vi "UHR-Fleezers Control (host) - 10.5.vi"() -> ()   [LabVIEW 2010] (continued)
    tunnel: "Initial Phase Adj. (MCL)" -> [w275]
    tunnel: w144 -> [w276]
    tunnel: w145 -> [w277]
    tunnel: "Initial Phase Adjustment (GI)" -> [w278]
    tunnel: "Initial Phase Adjustment (AI1)" -> [w279]
    tunnel: [w279] -> w8
    tunnel: [w278] -> w7
    tunnel: [w277] -> w6
    tunnel: [w276] -> w5
    tunnel: [w275] -> w4
    tunnel: [w274] -> w3
    tunnel: [w273] -> w2
    tunnel: [w291] -> w154
    tunnel: [w285] -> w150
    tunnel: "Initial Phase Adjustment (APD Acq)" -> [w284]
    tunnel: "Initial Phase Adjustment (APD 1 Gate)" -> [w283]
    tunnel: "Initial Phase Adjustment (Green FB)" -> [w282]
    tunnel: w8 -> [w290]
    tunnel: w7 -> [w289]
    tunnel: w6 -> [w288]
    tunnel: w5 -> [w287]
    tunnel: w4 -> [w286]
    tunnel: w3 -> [w281]
    tunnel: w2 -> [w280]
    tunnel: w154 -> [w470]
    tunnel: [w471] -> w151
    tunnel: w150 -> [w471]
    tunnel: [w470] -> w149
    tunnel: w151 -> [w474]
    tunnel: w149 -> [w473]
    tunnel: [w476] -> w148
    tunnel: [w475] -> w147
    tunnel: [w663] -> w152
    tunnel: [w664] -> w153
    tunnel: w148 -> [w664]
    tunnel: w147 -> [w663]
    frame #0 {
      n114 = Wait (ms)(milliseconds to wait=u32 200) -> ()  [unwired: 1 out]
    }
    frame #1 {
      n115 = xnode "Read/Write Control"("FPGA VI Reference In"=w288, "error in"=w287, "Phase count adjustment"=w290, "Phase count adjustment (GI)"=w289, "Phase count adjustment (MCL)"=w286, "Phase Count Adjustment (APD Acq)"=w284, "Phase count adjustment (APD 1 Gate)"=w283, "Phase count adjustment (APD 2 Gate)"=w280, "Phase count adjustment (Green FB)"=w282, "Phase count adjustment (GI) 2"=w281) -> ("FPGA VI Reference Out"=w285:T20, "error out"=w291:errorcluster)
    }
    frame #2 {
      n116 = Wait (ms)(milliseconds to wait=u32 200) -> ()  [unwired: 1 out]
    }
    frame #3 {
      w472 = TRUE
      n117 = xnode "Read/Write Control"("FPGA VI Reference In"=w474, "error in"=w473, "+ phase"=w472, "+ phase (GI)"=w472, "+ phase (MCL)"=w472, "+ phase (APD Acq)"=w472, "+ phase (APD 1 Gate)"=w472, "+ phase (APD 2 Gate)"=w472, "+ phase (Green FB)"=w472, "+ phase (GI) 2"=w472) -> ("FPGA VI Reference Out"=w475:T20, "error out"=w476:errorcluster)
    }
    frame #4 {
      n118 = Wait (ms)(milliseconds to wait=u32 200) -> ()  [unwired: 1 out]
    }
  }
  n119 = local read "Phase adj. (Green FB)"() -> (w118:i16)
  n120 = local read "Phase adj. (GI) 2"() -> (w88:i16)
  n121 = local read "Phase adjust (MCL)"() -> (w183:i16)
  n122 = local read "Phase adj. (AI1)"() -> (w185:i16)
  n123 = local read "Phase adj. (GI)"() -> (w184:i16)
  n124 = xnode "Read/Write Control"("FPGA VI Reference In"=w152, "error in"=w153, "Phase count adjustment"=w185, "Phase count adjustment (GI)"=w184, "Phase count adjustment (MCL)"=w183, "Phase Count Adjustment (APD Acq)"="Phase Adj. (APD Acq)", "Phase count adjustment (APD 1 Gate)"="Phase Adj. (APD 1 Gate)", "Phase count adjustment (APD 2 Gate)"="Phase Adj. (APD 2 Gate)", "Phase count adjustment (Green FB)"=w118, "Phase count adjustment (GI) 2"=w88) -> ("FPGA VI Reference Out"=w75:T20, "error out"=w161:errorcluster)
  n125 = call "Initialize RF boards - interlace 3.vi"("error in"=w161, "FPGA VI Reference In"=w75) -> ("error out"=w159:errorcluster, "FPGA VI Reference Out"=w160:T20)
  n126 = call "set RF board frequency - interlace.vi"("Board 2 Frequency Limits"=w121, "Board 1 Frequency Limits"=w123, "error in"=w159, "FPGA VI Reference In"=w160, "Board 2 Frequency 3 (MHz)"="BD 2 Frequency 3 (MHz)", "Board 1 Frequency 3 (MHz)"="BD 1 Frequency 3 (MHz)", "Board 2 Frequency 2 (MHz)"="BD 2 Frequency 2 (MHz)", "Board 2 Frequency 1 (MHz)"="BD 2 Frequency 1 (MHz)", "Board 1 Frequency 2 (MHz)"="BD 1 Frequency 2 (MHz)", "Board 1 Frequency 1  (MHz)"="BD 1 Frequency 1 (MHz)") -> ("error out"=w257:errorcluster, "FPGA VI Reference Out"=w258:T20)
  n127 = call "set RF board amplitude - interlace.vi"("Board 2 Amplitude Limits"=w120, "Board 1 Amplitude Limits"=w122, "error in"=w257, "FPGA VI Reference In"=w258, "Board 2 Amplitude 3 (%)"="BD 2 Amplitude 3 (%)", "Board 1 Amplitude 3 (%)"="BD 1 Amplitude 3 (%)", "Board 2 Amplitude 2 (%)"="BD 2 Amplitude 2 (%)", "Board 2 Amplitude 1 (%)"="BD 2 Amplitude 1 (%)", "Board 1 Amplitude 2 (%)"="BD 1 Amplitude 2 (%)", "Board 1 Amplitude 1 (%)"="BD 1 Amplitude 1 (%)") -> ("error out"=w245:errorcluster, "FPGA VI Reference Out"=w246:T20)
  n128 = flat-sequence {
    tunnel: w246 -> [w673]
    tunnel: w245 -> [w672]
    tunnel: [w671] -> w250
    tunnel: [w670] -> w249
    tunnel: [w715] -> w248
    tunnel: w250 -> [w715]
    tunnel: [w714] -> w247
    tunnel: w249 -> [w714]
    tunnel: w248 -> [w724]
    tunnel: w247 -> [w723]
    tunnel: [w722] -> w34
    tunnel: [w721] -> w33
    tunnel: [w780] -> w35
    tunnel: [w789] -> w9
    tunnel: w34 -> [w789]
    tunnel: w33 -> [w784]
    frame #0 {
      n129 = local read "Trap 1 (ON/OFF)"() -> (w665:bool)
      n130 = xnode "Read/Write Control"("FPGA VI Reference In"=w673, "error in"=w672, "Direct RF Box  Communication"=FALSE) -> ("FPGA VI Reference Out"=w671:T20, "error out"=w670:errorcluster)
      n131 = local write "Saving..."(FALSE ("Saving Data")) -> ()
      n132 = local write "Stop All"(FALSE ("Stop All")) -> ()
      n133 = local write "Index"(1.0 ("Index")) -> ()
      n134 = property on="Trap 1 ON" class="Bool (strict)"("Value"=w665) -> ()  [unwired: 2 in, 2 out]
      "Manipulating Trap" <- FALSE ("Manipulating Trap")
    }
    frame #1 {
      n135 = local read "Trap 2 (ON/OFF)"() -> (w713:bool)
      n136 = Wait (ms)(milliseconds to wait=u32 50) -> ()  [unwired: 1 out]
      n137 = property on="Trap 2 ON" class="Bool (strict)"("Val(Sgnl)"=w713) -> ()  [unwired: 2 in, 2 out]
    }
    frame #2 {
      n138 = local read "Scan Range (nm)"() -> (w717:dbl)
      n139 = xnode "Read/Write Control"("FPGA VI Reference In"=w724, "error in"=w723, "FPGA Controls  RF Box"=TRUE ("Direct RF Box  Communication")) -> ("FPGA VI Reference Out"=w722:T20, "error out"=w721:errorcluster)
      n140 = call "Update messages.vi"("Message to add"="UHR-Fleezers ready.", "Old message string"="") -> ("New message string"=w720:string)
      n141 = local write "Messages"(w720) -> ()
      n142 = property on="Scan Range (nm)" class="DigNum (strict)"("Val(Sgnl)"=w717) -> ()  [unwired: 2 in, 2 out]
    }
    frame #3 {
      w769 = T23."ASCII" ("Command")
      # "disable hysteresis\ncompensation for\nfaster performance"
      # "increase jerk\nfor faster \nresponse"
      # "disable backlash\ncompensation for\nfaster response \ntimes. necessary\nfor mouse control\nof stage"
      n143 = call "CONEX_FUNCTIONAL_GLOBAL.vi"("error in"=w784, "Command"=T23."INIT") -> ("error out"=w765:errorcluster)  [unwired: 7 in, 2 out]
      n144 = call "CONEX_FUNCTIONAL_GLOBAL.vi"("error in"=w765, "Position"=dbl[] [10.0, 12.0, 6.2], "Command"=T23."SET ULIM") -> ("error out"=w785:errorcluster)  [unwired: 6 in, 2 out]
      n145 = call "CONEX_FUNCTIONAL_GLOBAL.vi"("error in"=w785, "Position"=dbl[] [4.0, 0.0, 5.8], "Command"=T23."SET LLIM") -> ("error out"=w778:errorcluster)  [unwired: 6 in, 2 out]
      n146 = Concatenate Strings("1BA0", "\r\n") -> (w775:string)
      n147 = call "CONEX_FUNCTIONAL_GLOBAL.vi"("error in"=w778, "ASCII command"=w775, "Command"=w769) -> ("error out"=w774:errorcluster)  [unwired: 6 in, 2 out]
      n148 = Concatenate Strings("1JR0.001", "\r\n") -> (w771:string)
      n149 = call "CONEX_FUNCTIONAL_GLOBAL.vi"("error in"=w774, "ASCII command"=w771, "Command"=w769) -> ("error out"=w770:errorcluster)  [unwired: 6 in, 2 out]
      n150 = Concatenate Strings("1BH0", "\r\n") -> (w766:string)
      n151 = call "CONEX_FUNCTIONAL_GLOBAL.vi"("error in"=w770, "ASCII command"=w766, "Command"=w769) -> ("error out"=w764:errorcluster)  [unwired: 6 in, 2 out]
      n152 = call "CONEX_FUNCTIONAL_GLOBAL.vi"("error in"=w764, "Command"=T23."GET POS") -> ("error out"=w780:errorcluster, "Current Position"=w779:dbl[])  [unwired: 7 in, 1 out]
      n153 = local write "Current Position"(w779) -> ()
    }
  }
  n154 = Subtract(x="BD 1 Frequency 1 (MHz)", y="BD 1 Frequency 2 (MHz)") -> (x-y=w171:dbl)
  n155 = Subtract(x="BD 2 Frequency 1 (MHz)", y="BD 2 Frequency 2 (MHz)") -> (x-y=w170:dbl)
  n156 = Square(x=w170) -> (x^2=w168:dbl)
  n157 = Square(x=w171) -> (x^2=w169:dbl)
  n158 = Add(x=w169, y=w168) -> (x+y=w167:dbl)
  n159 = Square Root(x=w167) -> (sqrt(x)=w166:dbl)
  n160 = local write "Trap Delta (MHz)"(w166) -> ()
  n161 = call "IMAQ Create"("Image Name"="APD 1 Image", "Image Type"=w66) -> ("New Image"=w65:T2)  [unwired: 3 in, 1 out]
  n162 = call "IMAQ Create"("Image Name"="APD 2 Image", "Image Type"=w66) -> ("New Image"=w64:T2)  [unwired: 3 in, 1 out]
  n163 = call "IMAQ Create"("Image Name"="Det. X Image", "Image Type"=w66) -> ("New Image"=w63:T2)  [unwired: 3 in, 1 out]
  n164 = call "IMAQ Create"("Image Name"="Det. Y Image", "Image Type"=w66) -> ("New Image"=w62:T2)  [unwired: 3 in, 1 out]
  n165 = call-poly "VISA Configure Serial Port"("VISA resource name"="Harvard Syringe Pump Serial Port", "baud rate (9600)"=u32 115200, "stop bits (10: 1 bit)"=w59) -> ("VISA resource name out"=w56:refnum<visa-resource-name>, "error out"=w57:errorcluster)  [unwired: 4 in, 7 out]
  n166 = Bundle("New Image"=w65, "New Image"=w64, "New Image"=w63, "New Image"=w62) -> (w61:T24)  [unwired: 1 in]
  n167 = Tick Count (ms)() -> (millisecond timer value=w36:u32)
  n168 = call <vilib>:"IMAQ Init.vi"("Interface Name"="img0") -> ("error out"=w28:errorcluster, "IMAQ Session Out"=w30:refnum<k11>)  [unwired: 9 in]
  n169 = disable-structure shown="Disabled" {
    disable-tunnel: w9 -> [w792 _]
    frame Disabled {
      n170 = call <vilib>:"Initialize Mouse.vi"() -> ("device ID"=w791:refnum<k1>)  [unwired: 10 in, 1 out]
      n171 = while {
        tunnel: w792 -> [_]
        tunnel: w791 -> [w796]
        tunnel: [w795] -> w790
        stop <- w794 stop-if-true
        n172 = event shown="[2] \"Use mouse to move stage\n(press any key to quit)\": Value Change" {
          selector: _ -> [_ _ _ _]
          dyn-events: _ -> [_ _ _ _]
          timeout: 1 -> [_ _ _ _]
          tunnel: w796 -> [w797 w798 w808 _]
          tunnel: [w797 w798 w804 _] -> w795
          tunnel: [_ w799 _ _] -> w794
          event Timeout {
            n173 = event-data() -> ()  [unwired: 1 in, 2 out]
          }
          event "Stop All": Value Change {
            n174 = event-data() -> ()  [unwired: 1 in, 5 out]
            n175 = local read "Stop All"() -> (w799:bool)
          }
          event "Use mouse to move stage\n(press any key to quit)": Value Change {
            n176 = event-data() -> ()  [unwired: 1 in, 1 out]
            n177 = local write "Stage Moving"(TRUE ("Stage Moving")) -> ()
            n178 = call-poly <vilib>:"Acquire Input Data.vi"("device ID"=w808) -> ("device ID"=w805:refnum<k1>)  [unwired: 15 in, 3 out]
            n179 = node-c288() -> (w807:T25)  [unwired: 4 in]
            n180 = timed-loop {
              timing: w807 -> [_]
              timing-out: [_] -> w806
              tunnel: w805 -> [w838]
              tunnel: [w837] -> w804
              tunnel: [w810] -> w801
              stop <- w813 stop-if-true
              (unwired) 10
              # "put cursor somewhere\nwhere mouse clicks and \nmouse wheel moves won't\nbe heard by the window"
              # "SetCursorPos"
              n181 = node-c288() -> ()  [unwired: 1 in, 1 out]
              n182 = call-poly <vilib>:"Acquire Input Data.vi"("device ID"=w838, "key mode"=enum16{"RELATIVE", "ABSOLUTE"}."RELATIVE") -> ("device ID"=w837:refnum<k1>, "axis info"=w835:T28, "button info"=w825:T29)  [unwired: 14 in, 1 out]
              n183 = Cluster To Array(cluster=w835) -> (array=w833:i32[])
              n184 = Unbundle By Name(w825) -> ("button 1"=w824:bool, "button 2"=w823:bool, "button 3"=w822:bool)
              n185 = Compound Arithmetic op=MULTIPLY(invert 10000.0 ("value"), "mouse sensitivity", w833) -> (w831:dbl[])
              n186 = call "subVI_explode3array.vi"("Array"=w831) -> ("x"=w817:dbl, "y"=w816:dbl, "z"=w830:dbl)  [unwired: 12 in]
              n187 = case shown="False" "invert y?" {
                tunnel: w816 -> [w839 w841]
                tunnel: [w839 w840] -> w815
                frame False {
                }
                frame True {
                  n188 = Negate(x=w841) -> (-x=w840:dbl)
                }
              }
              n189 = case shown="False" "invert x?" {
                tunnel: w817 -> [w842 w844]
                tunnel: [w842 w843] -> w814
                frame False {
                }
                frame True {
                  n190 = Negate(x=w844) -> (-x=w843:dbl)
                }
              }
              n191 = Compound Arithmetic op=OR(w824, w823, w822) -> (w813:bool)
              n192 = Divide(x=w830, y=50.0) -> (x/y=w828:dbl)
              n193 = Build Array(w814, w815, w828) -> (w820:dbl[])
              n194 = Not(x=w813) -> (.not. x?=w821:bool)
              n195 = call "CONEX_FUNCTIONAL_GLOBAL.vi"("Axis"=enum16{"X", "Y", "Z", "XY", "XZ", "YZ", "XYZ"}."XYZ", "Position"=w820, "Command"=T23."REL MOVE") -> ("error out"=w810:errorcluster)  [unwired: 6 in, 2 out]
              n196 = dll-call lib="User32.dll" fn="SetCursorPos"(700, 45) -> ()  [unwired: 5 in, 3 out]
              n197 = local write "Stage Moving"(w821) -> ()
              n198 = node-c288() -> ()  [unwired: 1 in, 1 out]
            }
            n199 = node-c288(w806) -> ()  [unwired: 1 out]
            n200 = call "CONEX_FUNCTIONAL_GLOBAL.vi"("Axis"=enum16{"X", "Y", "Z", "XY", "XZ", "YZ", "XYZ"}."XYZ", "error in"=w801, "Command"=T23."GET POS") -> ("Current Position"=w800:dbl[])  [unwired: 6 in, 2 out]
            n201 = local write "Current Position"(w800) -> ()
          }
          event "reset motor comm. link": Value Change {
            n202 = event-data() -> ()  [unwired: 1 in, 1 out]
          }
        }
      }
      n203 = call-poly <vilib>:"Close Input Device.vi"("device ID"=w790) -> ()  [unwired: 9 in, 1 out]
    }
    frame Enabled {
    }
  }
  n204 = call <vilib>:"IMAQ Grab Setup.vi"("error in (no error)"=w28, "IMAQ Session In"=w30) -> ("error out"=w24:errorcluster, "IMAQ Session Out"=w25:refnum<k11>)  [unwired: 8 in]
  n205 = call "IMAQ Create"("Image Name"="untitled", "Image Type"=w26) -> ("New Image"=w23:T2)  [unwired: 3 in, 1 out]
  n206 = node-c288() -> (w32:T25)  [unwired: 4 in]
  n207 = timed-loop "acquire video and stage position" {
    timing: w32 -> [_]
    timing-out: [_] -> w31
    tunnel: w25 -> [w859]
    tunnel: w24 -> [w858]
    tunnel: w23 -> [w857]
    tunnel: [w856] -> w20
    tunnel: [w853] -> w19
    tunnel: [w854] -> w18
    tunnel: w9 -> [_]
    shift-right: [w850] -> _
    shift-left: cluster{i32, i32, i32, i32}[] [] -> [w851]
    stop <- w855 stop-if-true
    n208 = node-c288() -> ()  [unwired: 1 in, 1 out]
    n209 = event shown="[2] \"Primary Video Display\": Mouse Down" {
      selector: _ -> [_ _ _ _]
      dyn-events: _ -> [_ _ _ _]
      timeout: 10 -> [_ _ _ _]
      tunnel: w859 -> [w870 w885 w893 w913]
      tunnel: w858 -> [w869 w887 w891 w915]
      tunnel: w857 -> [w868 w886 w892 w914]
      tunnel: [w867 w885 w893 w913] -> w856
      tunnel: [w860 w889 FALSE FALSE] -> w855
      tunnel: [w864 w887 w891 w915] -> w854
      tunnel: [w863 w886 w892 w914] -> w853
      tunnel: "radius" -> [_ _ w899 _]
      tunnel: w851 -> [w861 w888 w897 _]
      tunnel: [w861 w888 w898 cluster{i32, i32, i32, i32}[] []] -> w850
      event Timeout {
        n210 = event-data() -> ()  [unwired: 1 in, 2 out]
        n211 = call <vilib>:"IMAQ Grab Acquire.vi"("error in (no error)"=w869, "Image In"=w868, "IMAQ Session In"=w870) -> ("error out"=w865:errorcluster, "Image Out"=w866:T2, "IMAQ Session Out"=w867:refnum<k11>)  [unwired: 5 in, 1 out]
        n212 = case shown="True" "trap\nmarkers?" {
          tunnel: w861 -> [_ w878]
          tunnel: w866 -> [w872 w877]
          tunnel: w865 -> [w871 w876]
          tunnel: [w871 w875] -> w864
          tunnel: [w872 w873] -> w863
          frame False {
          }
          frame True {
            n213 = for {
              tunnel: w878 -> [w884] mode=indexing
              shift-right: [w882] -> w873
              shift-left: w877 -> [w883]
              tunnel: w876 -> [w881]
              tunnel: [w880] -> w875
              tunnel: u32 16711680 ("Color") -> [w879]
              n214 = call "IMAQ Overlay Oval"("Color"=w879, "error in (no error)"=w881, "Bounding Rectangle"=w884, "Image"=w883) -> ("error out"=w880:errorcluster, "Image Out"=w882:T2)  [unwired: 6 in]
            }
          }
        }
        "Primary Video Display" <- w863
        n215 = Unbundle By Name(w865) -> ("status"=w860:bool)
      }
      event "Stop All": Value Change {
        n216 = event-data() -> ()  [unwired: 1 in, 5 out]
        n217 = local read "Stop All"() -> (w889:bool)
      }
      event "Primary Video Display": Mouse Down {
        n218 = event-data() -> ()  [unwired: 1 in, 7 out]
        n219 = Array Size(array=w897) -> (size(s)=w896:i32)
        n220 = Less?(x=w896, y=2) -> (x < y?=w894:bool)
        n221 = case shown="True" w894 {
          tunnel: w899 -> [_ w909]
          tunnel: w897 -> [w900 w903]
          tunnel: [w900 w902] -> w898
          frame False {
          }
          frame True {
            n222 = property on="Primary Video Display" class="ImageControl"() -> ("Last Mouse Position"=w901:cluster{"X":i32, "Y":i32})  [unwired: 2 in, 2 out]
            n223 = Unbundle By Name(w901) -> ("X"=w911:i32, "Y"=w910:i32)
            n224 = Add(x=w910, y=w909) -> (x+y=w907:i32)
            n225 = Subtract(x=w910, y=w909) -> (x-y=w905:i32)
            n226 = Add(x=w911, y=w909) -> (x+y=w906:i32)
            n227 = Subtract(x=w911, y=w909) -> (x-y=w908:i32)
            n228 = Bundle(w908, w907, w906, w905) -> (w904:cluster{i32, i32, i32, i32})  [unwired: 1 in]
            n229 = Build Array (concatenate)(w903, w904) -> (w902:cluster{i32, i32, i32, i32}[])
          }
        }
      }
      event "clear markers": Value Change {
        n230 = event-data() -> ()  [unwired: 1 in, 5 out]
      }
    }
    n231 = node-c288() -> ()  [unwired: 1 in, 1 out]
    "Array" <- w851
  }
  n232 = node-c288(i64 1 ("Period"), 1 ("Processor")) -> (w175:T25)  [unwired: 2 out]
  n233 = node-c288(2 ("Processor")) -> (w79:T25)  [unwired: 3 out]
  n234 = node-c288() -> (w71:T25)  [unwired: 4 in]
  n235 = node-c288() -> (w81:T25)  [unwired: 4 out]
  n236 = timed-loop "Acquire Data" {
    tunnel: w9 -> [w1175]
    tunnel: w35 -> [w1174]
    tunnel: [w1205] -> w11
    tunnel: [w1199] -> w10
    timing: w175 -> [_]
    timing-out: [_] -> w174
    tunnel: w61 -> [w1003]
    shift-right: [w920] -> _
    shift-left: w36 -> [w922]
    stop <- "Stop All" stop-if-true
    (unwired) u32 0 ("Number of Elements")
    w990 = "NI_ChannelName" ("name")
    # "originally this was Trap AI FIFO Depth -\nTrap AI Elements/DMA read. The subtraction\nof zero is a kluge to make it work."
    n237 = node-c288() -> ()  [unwired: 2 out]
    n238 = Tick Count (ms)() -> (millisecond timer value=w920:u32)
    n239 = First Call?() -> (First Call?: T/F=w956:bool)
    n240 = Subtract(x=w920, y=w922) -> (x-y=→"x-y":u32)
    n241 = Or(x="Reset", y=w956) -> (x .or. y?=w957:bool)
    n242 = case "Reset data stream" shown="True" w957 {
      tunnel: w1175 -> [w1219 w1227]
      tunnel: w1174 -> [w1218 w1226]
      tunnel: [w1219 w1221] -> w1170
      tunnel: [w1218 w1220] -> w1169
      frame False {
      }
      frame True {
        w1224 = TRUE ("AI to FIFO")
        n243 = local write "Overflow (data lost)"(FALSE ("Overflow (data lost)")) -> ()
        n244 = call "reset FPGA DMA.vi"("error in"=w1226, "FPGA VI Reference In"=w1227) -> ("error out"=w1222:errorcluster, "FPGA VI Reference Out"=w1223:T20)
        n245 = xnode "Read/Write Control"("FPGA VI Reference In"=w1223, "error in"=w1222, "AI to FIFO"=w1224, "APD to FIFO"=w1224) -> ("FPGA VI Reference Out"=w1221:T20, "error out"=w1220:errorcluster)
      }
    }
    n246 = Or(x="Start AOD Scan", y="Trap Raster Scan") -> (x .or. y?=w1120:bool)
    n247 = case "Start AOM raster scan" shown="False" w1120 {
      tunnel: w1170 -> [w2835 w2845]
      tunnel: w1169 -> [w2834 w2844]
      tunnel: [w2835 w2838] -> w1168
      tunnel: [w2834 w2837] -> w1167
      frame False {
      }
      frame True {
        n248 = case shown="True" "Restart DMA? (AOD)" {
          tunnel: [w3256 w3258] -> w2839
          tunnel: [w3255 w3257] -> w2840
          tunnel: w2845 -> [w3256 w3260]
          tunnel: w2844 -> [w3255 w3259]
          frame False {
          }
          frame True {
            n249 = local write "Overflow (data lost)"(FALSE ("Overflow (data lost)")) -> ()
            n250 = call "reset FPGA DMA.vi"("error in"=w3259, "FPGA VI Reference In"=w3260) -> ("error out"=w3257:errorcluster, "FPGA VI Reference Out"=w3258:T20)
          }
        }
        n251 = local write "Trap Raster Scan"(FALSE ("Trap Raster Scan")) -> ()
        n252 = case shown="True" "Move MCL Also?" {
          tunnel: w2840 -> [w2848 w2957]
          tunnel: w2839 -> [w2849 w2958]
          tunnel: [w2847 w2961] -> w2838
          tunnel: [w2846 w2960] -> w2837
          frame False {
            w2850 = TRUE ("AI to FIFO")
            n253 = xnode "Read/Write Control"("FPGA VI Reference In"=w2849, "error in"=w2848, "AI to FIFO"=w2850, "APD to FIFO"=w2850, "Start scan"=w2850) -> ("FPGA VI Reference Out"=w2847:T20, "error out"=w2846:errorcluster)
          }
          frame True {
            w2954 = FALSE ("1D or 2D Scan?")
            w2959 = TRUE ("AI to FIFO")
            # "Count for MCL loop"
            # "N total cycles"
            # "N steps"
            # "V_int"
            n254 = local read "Scan Range (nm)"() -> (w2936:dbl)
            n255 = local read "Number of F/B Scans (AOD)"() -> (w2953:u16)
            n256 = Sign(1:w2936) -> (0:w2935:dbl)
            n257 = Compound Arithmetic op=MULTIPLY(w2936, "MCL Step Position Ratio", "MCL/AOM Scale Tweak") -> (w2940:dbl)
            n258 = Negate(x=w2935) -> (-x=w2932:dbl)
            n259 = Multiply(x=w2932, y="MCL Step Increment (V_int)") -> (x*y=w2934:dbl)
            n260 = Divide(x=w2940, y="MCL X Cal (nm/V)") -> (x/y=w2946:dbl)
            n261 = Multiply(x=32767.0 ("y"), y=w2946) -> (x*y=w2952:dbl)
            n262 = local read "Total Counts (ticks)"() -> (w2937:u32)
            n263 = local read "Cycles/step (AOD)"() -> (w2948:u64)
            n264 = local read "Scan steps (AOD)"() -> (w2949:u64)
            n265 = Divide(x=w2952, y=10.0) -> (x/y=w2945:dbl)
            n266 = Divide(x=w2945, y="MCL Step Increment (V_int)") -> (x/y=w2943:dbl)
            n267 = Absolute Value(x=w2943) -> (abs(x)=w2931:dbl)
            n268 = Compound Arithmetic op=MULTIPLY(w2949, w2948, w2937) -> (w2944:u64)
            n269 = local write "wait to reset values"(w2959) -> ()
            n270 = local write "MCL Scanning"(w2959) -> ()
            n271 = Divide(x=w2944, y=w2931) -> (x/y=w2941:dbl)
            "MCL Count" <- w2941
            n272 = xnode "Read/Write Control"("FPGA VI Reference In"=w2958, "error in"=w2957, "Scan steps (MCL)"=w2931, "Number of scans (MCL)"=w2953, "Cycles per step (MCL)"=u64 1, "Scan freq.  increment (MCL)"=w2934, "1D or 2D Scan?"=w2954, "MCL Scan Axis"=w2954, "Cont. Scan (MCL)"=w2954, "MCL count"=w2941) -> ("FPGA VI Reference Out"=w2956:T20, "error out"=w2955:errorcluster)
            n273 = xnode "Read/Write Control"("FPGA VI Reference In"=w2956, "error in"=w2955, "AI to FIFO"=w2959, "APD to FIFO"=w2959, "Start scan"=w2959, "Start scan (MCL)"=w2959) -> ("FPGA VI Reference Out"=w2961:T20, "error out"=w2960:errorcluster)
          }
        }
        "Raster Scanning..." <- TRUE ("Scanning...")
      }
    }
    n274 = And(x="Save scans", y=w1120) -> (x .and. y?=w1166:bool)
    n275 = Compound Arithmetic op=OR("Start MCL Scan", "Confocal Image", "Confocal Linescan") -> (w1118:bool)
    n276 = And(x="Save Data (MCL)", y=w1118) -> (x .and. y?=w1165:bool)
    n277 = case "Start MCL raster scan" shown="False" w1118 {
      tunnel: w1168 -> [w2176 w2191]
      tunnel: w1167 -> [w2175 w2190]
      tunnel: [w2176 w2186] -> w924
      tunnel: [w2175 w2185] -> w923
      tunnel: [FALSE w2184] -> w1151
      tunnel: "Start MCL Scan" -> [_ w2179]
      tunnel: "Confocal Image" -> [_ w2178]
      tunnel: "Confocal Linescan" -> [_ _]
      frame False {
      }
      frame True {
        w2184 = TRUE
        n278 = case shown="True" "Restart DMA? (MCL)" {
          tunnel: [w2436 w2438] -> w2189
          tunnel: [w2435 w2437] -> w2188
          tunnel: w2191 -> [w2436 w2441]
          tunnel: w2190 -> [w2435 w2440]
          frame False {
          }
          frame True {
            n279 = call "reset FPGA DMA.vi"("error in"=w2440, "FPGA VI Reference In"=w2441) -> ("error out"=w2437:errorcluster, "FPGA VI Reference Out"=w2438:T20)
            n280 = local write "Overflow (data lost)"(FALSE ("Overflow (data lost)")) -> ()
          }
        }
        n281 = case shown="False" w2179 {
          selector: w2179 -> [_ w2195]
          tunnel: w2178 -> [w2194 _]
          tunnel: [w2194 w2195] -> w2177
          frame False {
            n282 = property on="2D or 1D Scan" class="Bool (strict)"("Val(Sgnl)"=w2194) -> ()  [unwired: 2 in, 2 out]
            n283 = property on="Confocal Image" class="Bool (strict)"("Value"=FALSE ("Start Confocal Map")) -> ()  [unwired: 2 in, 2 out]
          }
          frame True {
          }
        }
        n284 = local write "MCL Scanning"(w2184) -> ()
        n285 = local read "AO1"() -> (w2181:dbl)
        n286 = local read "AO2"() -> (w2180:dbl)
        n287 = case shown="False" "Center Scan" {
          tunnel: w2189 -> [w2202 w2314]
          tunnel: w2188 -> [w2201 w2313]
          tunnel: [w2200 w2312] -> w2186
          tunnel: [w2199 w2311] -> w2185
          tunnel: [w2197 w2298] -> w2183
          tunnel: [w2196 w2297] -> w2182
          tunnel: w2181 -> [w2197 w2303]
          tunnel: w2180 -> [w2196 w2306]
          tunnel: w2177 -> [_ _]
          frame False {
            w2198 = TRUE ("AI to FIFO")
            n288 = xnode "Read/Write Control"("FPGA VI Reference In"=w2202, "error in"=w2201, "AI to FIFO"=w2198, "APD to FIFO"=w2198, "Start scan (MCL)"=w2198) -> ("FPGA VI Reference Out"=w2200:T20, "error out"=w2199:errorcluster)
          }
          frame True {
            w2310 = TRUE ("AI to FIFO")
            n289 = local read "Scan steps (MCL)"() -> (w2289:u64)
            n290 = local read "Scan lines (y)"() -> (w2285:u64)
            n291 = local read "Fast Scan Dir"() -> (w2296:bool)
            n292 = local read "Actual MCL Inc (V)"() -> (w2286:dbl)
            n293 = Decrement(x=w2285) -> (x-1=w2284:u64)
            n294 = Decrement(x=w2289) -> (x-1=w2288:u64)
            n295 = Multiply(x=w2286, y=w2284) -> (x*y=w2283:dbl)
            n296 = Divide(x=w2283, y=2.0) -> (x/y=w2293:dbl)
            n297 = Multiply(x=w2286, y=w2288) -> (x*y=w2287:dbl)
            n298 = Divide(x=w2287, y=2.0) -> (x/y=w2292:dbl)
            n299 = Select(t=w2292, s=w2296, f=w2293) -> (s? t:f=w2291:dbl)
            n300 = Select(t=w2293, s=w2296, f=w2292) -> (s? t:f=w2295:dbl)
            n301 = Subtract(x=w2303, y=w2295) -> (x-y=w2294:dbl)
            n302 = Subtract(x=w2306, y=w2291) -> (x-y=w2290:dbl)
            n303 = local read "2D or 1D Scan"() -> (w2308:bool)
            n304 = Not(x=w2296) -> (.not. x?=w2302:bool)
            n305 = Not(x=w2308) -> (.not. x?=w2304:bool)
            n306 = And(x=w2296, y=w2304) -> (x .and. y?=w2305:bool)
            n307 = And(x=w2304, y=w2302) -> (x .and. y?=w2307:bool)
            n308 = Select(t=w2306, s=w2307, f=w2290) -> (s? t:f=w2297:dbl)
            n309 = Select(t=w2303, s=w2305, f=w2294) -> (s? t:f=w2298:dbl)
            n310 = call "Volt to I16.vi"("Voltage In"=w2298) -> ("I16 Voltage Out"=w2301:i16)
            n311 = call "Volt to I16.vi"("Voltage In"=w2297) -> ("I16 Voltage Out"=w2300:i16)
            n312 = xnode "Read/Write Control"("FPGA VI Reference In"=w2314, "error in"=w2313, "AI to FIFO"=w2310, "APD to FIFO"=w2310, "Start scan (MCL)"=w2310, "AO1"=w2301, "AO2"=w2300) -> ("FPGA VI Reference Out"=w2312:T20, "error out"=w2311:errorcluster)
          }
        }
        "Initial Y" <- w2183
        "Initial X" <- w2182
        "wait to reset values" <- w2184
      }
    }
    n313 = local read "Trap Pos Elements/DMA read"() -> (w999:u32)
    n314 = local read "Trap AI Elements/DMA read"() -> (w919:u32)
    n315 = local read "APD Elements/DMA read"() -> (w1042:u32)
    n316 = local read "Trap AI FIFO Depth"() -> (w1215:u32)
    n317 = xnode "Get APD Data"("FPGA VI Reference In"=w924, "error in"=w923, "Number of Elements"=w1042, "Timeout (ms)"=-1) -> ("Data"=w1041:u32[], "Elements Remaining"=→"APD FIFO Elements Remaining":u32)  [unwired: 2 out]
    n318 = xnode "Invoke Method"("FPGA VI Reference In"=w924, "error in"=w923, "Number of Elements"=w999, "Timeout (ms)"=-1) -> ("Data"=w963:u16[], "Elements Remaining"=→"Trap Pos FIFO El Remaining":u32)  [unwired: 2 out]
    n319 = xnode "Invoke Method"("FPGA VI Reference In"=w924, "error in"=w923, "Number of Elements"=w919, "Timeout (ms)"=-1 ("Timeout")) -> ("FPGA VI Reference Out"=w926:T20, "error out"=w925:errorcluster, "Data"=w928:i16[], "Elements Remaining"=w927:u32)
    "Trap AI FIFO El. Rem." <- w927
    n320 = Subtract(x=w1215, y=w919) -> (x-y=w1214:u32)
    n321 = Decimate 1D Array(w963) -> (w960:u16[], w962:u16[], w961:u16[])
    n322 = Divide(x=w927, y=w1214) -> (x/y=w1213:dbl)
    "Buffer Status" <- w1213
    n323 = To Unsigned Long Integer(number=w960) -> (unsigned 32bit integer=w959:u32[])
    n324 = Join Numbers(hi=w962, lo=w961) -> ((hi.lo)=w958:u32[])
    n325 = Equal?(x=w1213, y=1.0) -> (x = y?=w1211:bool)
    n326 = Join Numbers(hi=w959, lo=w958) -> ((hi.lo)=w952:u64[])
    n327 = call "IR AOM word to freq - vec.vi"("Frequency Word In (double vec)"=w952) -> ("Frequency Out"=w998:dbl[])
    n328 = case "Alert buffer overflow" shown="True" w1211 {
      frame False {
      }
      frame True {
        n329 = call <vilib>:"Beep.vi"() -> ()  [unwired: 3 in, 9 out]
        "Overflow (data lost)" <- TRUE ("Overflow (data lost)")
      }
    }
    n330 = Decimate 1D Array(w998) -> (w997:dbl[], w996:dbl[])
    n331 = Build Array(w997, w996) -> (w995:dbl[][])
    n332 = local read "Trap Sets"() -> (w1079:u32)
    n333 = case "Deinterlace trap data, average down PSD" shown="2" w1079 {
      tunnel: w928 -> [w2471 w2536]
      tunnel: [w2468 w2533] -> w1072
      tunnel: [w2471 w2535] -> w955
      tunnel: "Detector Type" -> [w2470 w2531]
      tunnel: [w2469 w2534] -> w1071
      tunnel: [w2467 w2532] -> w1186
      frame 1, Default {
        n334 = Divide(x=w2471, y=3276.7) -> (x/y=w2472:dbl[])
        n335 = Decimate 1D Array(w2472) -> (w2481:dbl[], w2480:dbl[], w2479:dbl[], w2478:dbl[], w2477:dbl[], w2476:dbl[], w2475:dbl[], w2474:dbl[])
        n336 = case shown="\"IR-QPD + PSD + FB-QPD position\"" w2470 {
          tunnel: w2481 -> [w2505 w2530]
          tunnel: w2480 -> [w2504 w2529]
          tunnel: w2479 -> [w2489 w2507]
          tunnel: w2478 -> [w2490 w2517]
          tunnel: w2477 -> [w2503 w2528]
          tunnel: w2476 -> [w2502 w2527]
          tunnel: w2475 -> [w2486 w2508]
          tunnel: w2474 -> [w2485 w2506]
          tunnel: [w2484 w2514] -> w2469
          tunnel: [w2483 w2513] -> w2468
          tunnel: [w2482 w2512] -> w2467
          frame "IR-QPD + PSD + FB-QPD", Default {
            w2482 = 0  # Channel pattern
            n337 = Divide(x=w2505, y=w2490) -> (x/y=w2492:dbl[])
            n338 = Divide(x=w2504, y=w2490) -> (x/y=w2491:dbl[])
            n339 = Divide(x=w2503, y=w2486) -> (x/y=w2488:dbl[])
            n340 = Divide(x=w2502, y=w2485) -> (x/y=w2487:dbl[])
            n341 = Build Array(w2492, w2491, w2490, w2489, w2488, w2487, w2486, w2485) -> (w2483:dbl[][])
            n342 = Bundle("T1 Y", "T1 X", "T1 Sum", "FB Sum", "PSD Y", "PSD X", "PSD Y Sum", "PSD X Sum") -> (w2501:T39)  [unwired: 1 out]
            n343 = Cluster To Array(cluster=w2501) -> (array=w2484:string[])
          }
          frame "IR-QPD + PSD + FB-QPD position" {
            w2512 = 3  # Channel pattern
            n344 = Negate(x=w2508) -> (-x=w2509:dbl[])
            n345 = Divide(x=w2530, y=w2517) -> (x/y=w2519:dbl[])
            n346 = Divide(x=w2529, y=w2517) -> (x/y=w2518:dbl[])
            n347 = Divide(x=w2528, y=w2508) -> (x/y=w2516:dbl[])
            n348 = Divide(x=w2527, y=w2509) -> (x/y=w2515:dbl[])
            n349 = Build Array(w2519, w2518, w2517, w2506, w2507, w2516, w2515, w2508) -> (w2513:dbl[][])
            n350 = Bundle("T1 Y", "T1 X", "T1 Sum", "FB X", "FB Sum", "PSD Y", "PSD X", "PSD Y Sum") -> (w2526:T39)  [unwired: 1 out]
            n351 = Cluster To Array(cluster=w2526) -> (array=w2514:string[])
          }
        }
      }
      frame 2 {
        n352 = case shown="\"IR-QPD + PSD + FB-QPD X position\"" w2531 {
          tunnel: w2536 -> [w2598 w2665 w2736]
          tunnel: [w2537 w2656 w2667] -> w2535
          tunnel: [w2564 w2647 w2714] -> w2534
          tunnel: [w2563 w2610 w2681] -> w2533
          tunnel: [w2557 w2645 w2712] -> w2532
          frame "IR-QPD + PSD + FB-QPD", Default {
            w2557 = 1  # Channel pattern
            # "time average x2 the 4th signal and the 4 psd signals (detection laser)"
            # "deinterlace 3 signals from qpd"
            n353 = Decimate 1D Array(w2598) -> (w2597:i16[], w2596:i16[], w2562:i16[], w2595:i16[], w2585:i16[], w2583:i16[], w2582:i16[], w2580:i16[])
            n354 = Decimate 1D Array(w2562) -> (w2561:i16[], w2560:i16[])
            n355 = Decimate 1D Array(w2597) -> (w2594:i16[], w2566:i16[])
            n356 = Decimate 1D Array(w2596) -> (w2593:i16[], w2591:i16[])
            n357 = Decimate 1D Array(w2595) -> (w2592:i16[], w2590:i16[])
            n358 = call "downsample 1D array - double.vi"("Ave N"=2.0, "Array In"=w2585) -> ("Array Out"=w2584:dbl[])  [unwired: 1 out]
            n359 = call "downsample 1D array - double.vi"("Ave N"=2.0, "Array In"=w2583) -> ("Array Out"=w2565:dbl[])  [unwired: 1 out]
            n360 = call "downsample 1D array - double.vi"("Ave N"=2.0, "Array In"=w2582) -> ("Array Out"=w2581:dbl[])  [unwired: 1 out]
            n361 = call "downsample 1D array - double.vi"("Ave N"=2.0, "Array In"=w2580) -> ("Array Out"=w2579:dbl[])  [unwired: 1 out]
            n362 = Interleave 1D Arrays(w2594, w2593, w2592, w2566, w2591, w2590, w2561, w2560, w2584, w2565, w2581, w2579) -> (w2578:dbl[])
            n363 = Divide(x=w2578, y=3276.7) -> (x/y=w2577:dbl[])
            n364 = Decimate 1D Array(w2577) -> (w2576:dbl[], w2575:dbl[], w2574:dbl[], w2573:dbl[], w2572:dbl[], w2571:dbl[], w2559:dbl[], w2558:dbl[], w2570:dbl[], w2569:dbl[], w2568:dbl[], w2567:dbl[])
            n365 = Divide(x=w2576, y=w2574) -> (x/y=w2544:dbl[])
            n366 = Divide(x=w2575, y=w2574) -> (x/y=w2543:dbl[])
            n367 = Divide(x=w2573, y=w2571) -> (x/y=w2542:dbl[])
            n368 = Divide(x=w2572, y=w2571) -> (x/y=w2541:dbl[])
            n369 = Divide(x=w2570, y=w2568) -> (x/y=w2540:dbl[])
            n370 = Divide(x=w2569, y=w2567) -> (x/y=w2539:dbl[])
            n371 = Build Array(w2544, w2543, w2574, w2542, w2541, w2571, w2559, w2558, w2540, w2539, w2568, w2567) -> (w2563:dbl[][])
            n372 = Bundle("T1 Y", "T1 X", "T1 Sum", "T2 Y", "T2 X", "T2 Sum", "T1 FB Sum", "T2 FB Sum", "PSD Y", "PSD X", "PSD Y Sum", "PSD X Sum") -> (w2545:T40)  [unwired: 1 out]
            n373 = To Word Integer(number=w2578) -> (16bit integer=w2537:i16[])
            n374 = Cluster To Array(cluster=w2545) -> (array=w2564:string[])
          }
          frame "IR-QPD + PSD + FB-QPD X position" {
            w2645 = 2  # Channel pattern
            # "time average x2 the 3 psd signals (detection laser)"
            # "deinterlace 3 signals from qpds"
            n375 = Decimate 1D Array(w2665) -> (w2664:i16[], w2663:i16[], w2646:i16[], w2662:i16[], w2608:i16[], w2605:i16[], w2602:i16[], w2633:i16[])
            n376 = Decimate 1D Array(w2646) -> (w2631:i16[], w2629:i16[])
            n377 = Decimate 1D Array(w2664) -> (w2661:i16[], w2648:i16[])
            n378 = Decimate 1D Array(w2663) -> (w2660:i16[], w2658:i16[])
            n379 = Decimate 1D Array(w2662) -> (w2659:i16[], w2657:i16[])
            n380 = Decimate 1D Array(w2633) -> (w2632:i16[], w2630:i16[])
            n381 = call "downsample 1D array - I16.vi"("Ave N"=2.0, "Array In"=w2608) -> ("Array Out"=w2606:i16[])  [unwired: 1 in]
            n382 = call "downsample 1D array - I16.vi"("Ave N"=2.0, "Array In"=w2602) -> ("Array Out"=w2600:i16[])  [unwired: 1 in]
            n383 = call "downsample 1D array - I16.vi"("Ave N"=2.0, "Array In"=w2605) -> ("Array Out"=w2603:i16[])  [unwired: 1 in]
            n384 = Interleave 1D Arrays(w2661, w2660, w2659, w2648, w2658, w2657, w2632, w2631, w2630, w2629, w2606, w2603, w2600) -> (w2656:i16[])
            n385 = Divide(x=w2656, y=3276.7) -> (x/y=w2655:dbl[])
            n386 = Decimate 1D Array(w2655) -> (w2654:dbl[], w2653:dbl[], w2652:dbl[], w2651:dbl[], w2650:dbl[], w2649:dbl[], w2621:dbl[], w2619:dbl[], w2618:dbl[], w2616:dbl[], w2615:dbl[], w2614:dbl[], w2611:dbl[])
            n387 = Negate(x=w2611) -> (-x=w2609:dbl[])
            n388 = Divide(x=w2615, y=w2611) -> (x/y=w2613:dbl[])
            n389 = Divide(x=w2614, y=w2609) -> (x/y=w2612:dbl[])
            n390 = Divide(x=w2654, y=w2652) -> (x/y=w2637:dbl[])
            n391 = Divide(x=w2653, y=w2652) -> (x/y=w2636:dbl[])
            n392 = Divide(x=w2651, y=w2649) -> (x/y=w2635:dbl[])
            n393 = Divide(x=w2650, y=w2649) -> (x/y=w2634:dbl[])
            n394 = Divide(x=w2621, y=w2619) -> (x/y=w2620:dbl[])
            n395 = Divide(x=w2618, y=w2616) -> (x/y=w2617:dbl[])
            n396 = Build Array(w2637, w2636, w2652, w2635, w2634, w2649, w2620, w2619, w2617, w2616, w2613, w2612, w2611) -> (w2610:dbl[][])
            n397 = Bundle("T1 Y", "T1 X", "T1 Sum", "T2 Y", "T2 X", "T2 Sum", "T1 FB X", "T1 FB Sum", "T2 FB X", "T2 FB Sum", "PSD Y", "PSD X", "PSD Y Sum") -> (w2638:T41)  [unwired: 1 out]
            n398 = Cluster To Array(cluster=w2638) -> (array=w2647:string[])
          }
          frame "IR-QPD + PSD + FB-QPD XY positions" {
            w2712 = 4  # Channel pattern
            # "time average x2 the 3 psd signals (detection laser)"
            # "deinterlace 3 signals from qpds"
            n399 = Decimate 1D Array(w2736) -> (w2735:i16[], w2734:i16[], w2713:i16[], w2733:i16[], w2679:i16[], w2725:i16[], w2724:i16[], w2701:i16[])
            n400 = Decimate 1D Array "Feedback Sum"(w2713) -> (w2697:i16[], w2695:i16[])
            n401 = Decimate 1D Array "QPD Y"(w2735) -> (w2732:i16[], w2715:i16[])
            n402 = Decimate 1D Array "QPD X"(w2734) -> (w2731:i16[], w2729:i16[])
            n403 = Decimate 1D Array "Feedback Y"(w2679) -> (w2678:i16[], w2677:i16[])
            n404 = Decimate 1D Array "QPD Sum"(w2733) -> (w2730:i16[], w2728:i16[])
            n405 = Decimate 1D Array "Feedback X"(w2701) -> (w2698:i16[], w2696:i16[])
            n406 = call "downsample 1D array - double.vi"("Ave N"=2.0, "Array In"=w2725) -> ("Array Out"=w2700:dbl[])  [unwired: 1 out]
            n407 = call "downsample 1D array - double.vi"("Ave N"=2.0, "Array In"=w2724) -> ("Array Out"=w2699:dbl[])  [unwired: 1 out]
            n408 = Interleave 1D Arrays(w2732, w2731, w2730, w2715, w2729, w2728, w2678, w2698, w2697, w2677, w2696, w2695, w2700, w2699) -> (w2723:dbl[])
            n409 = Divide(x=w2723, y=3276.7) -> (x/y=w2722:dbl[])
            n410 = Decimate 1D Array(w2722) -> (w2721:dbl[], w2720:dbl[], w2719:dbl[], w2718:dbl[], w2717:dbl[], w2716:dbl[], w2674:dbl[], w2688:dbl[], w2672:dbl[], w2673:dbl[], w2686:dbl[], w2670:dbl[], w2684:dbl[], w2682:dbl[])
            n411 = Negate(x=w2682) -> (-x=w2680:dbl[])
            n412 = Divide(x=w2684, y=w2680) -> (x/y=w2683:dbl[])
            n413 = Divide(x=w2673, y=w2670) -> (x/y=w2669:dbl[])
            n414 = Divide(x=w2674, y=w2672) -> (x/y=w2671:dbl[])
            n415 = Divide(x=w2721, y=w2719) -> (x/y=w2705:dbl[])
            n416 = Divide(x=w2720, y=w2719) -> (x/y=w2704:dbl[])
            n417 = Divide(x=w2718, y=w2716) -> (x/y=w2703:dbl[])
            n418 = Divide(x=w2717, y=w2716) -> (x/y=w2702:dbl[])
            n419 = Divide(x=w2688, y=w2672) -> (x/y=w2687:dbl[])
            n420 = Divide(x=w2686, y=w2670) -> (x/y=w2685:dbl[])
            n421 = Build Array(w2705, w2704, w2719, w2703, w2702, w2716, w2671, w2687, w2672, w2669, w2685, w2670, w2683, w2682) -> (w2681:dbl[][])
            n422 = Bundle("T1 Y", "T1 X", "T1 Sum", "T2 Y", "T2 X", "T2 Sum", "T1 FB Y", "T1 FB X", "T1 FB Sum", "T2 FB Y", "T2 FB X", "T2 FB Sum", "PSD X", "PSD Y Sum") -> (w2668:T42)  [unwired: 1 out]
            n423 = To Word Integer(number=w2723) -> (16bit integer=w2667:i16[])
            n424 = Cluster To Array(cluster=w2668) -> (array=w2714:string[])
          }
        }
      }
    }
    "AI labels" <- w1071
    n425 = Decimate 1D Array(w1041) -> (w1069:u32[], w1005:u32[])
    n426 = local read "DMA Update Period (s)"() -> (w1080:dbl)
    n427 = local read "BD 1 Frequency 2 (MHz)"() -> (w947:dbl)
    n428 = local read "BD 1 Frequency 1 (MHz)"() -> (w948:dbl)
    n429 = Build Array(w1069, w1005) -> (w1148:u32[][])
    n430 = local read "Data Period (s)"() -> (w1054:dbl)
    n431 = Decimate 1D Array(w955) -> (w978:i16[], w977:i16[], w975:i16[], w974:i16[])  [unwired: 9 out]
    n432 = To Double Precision Float(number=w1148) -> (double precision float=w1149:dbl[][])
    n433 = local read "APD Integration Time (s)"() -> (w1018:dbl)
    n434 = Divide(x=w978, y=w977) -> (x/y=w979:dbl[])
    n435 = Divide(x=w975, y=w974) -> (x/y=w976:dbl[])
    n436 = feedback #1(0.0) -> (w992:dbl)
    n437 = Add(x=w1080, y=w992) -> (x+y=w1188:dbl)
    n438 = feedback-in #1(w1188) -> ()
    n439 = local read "AOM X Cal (nm/MHz)"() -> (w945:dbl)
    n440 = To Time Stamp(1:w992) -> (0:w991:timestamp)
    n441 = Split 1D Array(array=w979, index="N El. to Ave.") -> (second subarray=w982:dbl[])  [unwired: 1 out]
    n442 = Split 1D Array(array=w976, index="N El. to Ave.") -> (second subarray=w981:dbl[])  [unwired: 1 out]
    n443 = local read "Trap X AI1 (DMA)"() -> (w980:T14)
    n444 = Multiply(x=w1054, y="Trap Disp. Downsample") -> (x*y=w993:dbl)
    "Display Period (s)" <- w993
    n445 = Bundle("BD 1 Frequency 1 (MHz)"=w948, "BD 1 Frequency 2 (MHz)"=w947) -> (w949:T43)  [unwired: 1 out]
    n446 = for "Trap AI" {
      tunnel: [w2466] -> w1182 mode=indexing
      tunnel: w991 -> [w2456]
      tunnel: "Trap Disp. Downsample" -> [w2464]
      tunnel: w1072 -> [w2462] mode=indexing
      tunnel: w1054 -> [w2461]
      tunnel: w1071 -> [w2460] mode=indexing
      tunnel: w990 -> [w2459]
      tunnel: [w2458] -> w1029 mode=indexing
      tunnel: w993 -> [w2457]
      workers-P: _ -> [_]
      n447 = Bundle By Name("Y"=w2462, "dt"=w2461) -> (w2463:waveform(dbl))  [unwired: 1 out]
      n448 = Set Waveform Attribute(5:w2460, 6:w2459, 7:w2463) -> (3:w2458:waveform(dbl))  [unwired: 1 in, 2 out]
      n449 = call "downsample 1D array - double.vi"("Ave N"=w2464, "Array In"=w2462) -> ("Array Out"=w2465:dbl[])  [unwired: 1 out]
      n450 = Bundle By Name(cluster=w2458, "t0"=w2456, "Y"=w2465, "dt"=w2457) -> (w2466:waveform(dbl))
    }
    n451 = call <vilib>:"Mean.vi"("X"=w981) -> ("mean"=w969:dbl)  [unwired: 1 out]
    n452 = call <vilib>:"Mean.vi"("X"=w982) -> ("mean"=w970:dbl)  [unwired: 1 out]
    n453 = Cluster To Array(cluster=w949) -> (array=w946:dbl[])
    n454 = Reciprocal(x=w993) -> (1/x=→"Trap Disp. Freq. (Hz)":dbl)
    n455 = local read "Data points/scans (MCL)"() -> (w1160:dbl)
    n456 = To Fixed-Point(number=w969) -> (fixed-point=w967:fxp<+/-,16,1>)  [unwired: 1 in]
    n457 = To Fixed-Point(number=w970) -> (fixed-point=w968:fxp<+/-,16,1>)  [unwired: 1 in]
    n458 = Bundle("Trap 1 Pos.", "Trap 2 Pos.") -> (w989:cluster{string, string})  [unwired: 1 out]
    n459 = Bundle By Name(cluster=w980, "Set 1"=w968, "Set 2"=w967) -> (→"Trap X AI1 (DMA)":T14)
    n460 = Cluster To Array(cluster=w989) -> (array=w986:string[])
    n461 = for "Trap Position" {
      tunnel: w995 -> [w1371] mode=indexing
      tunnel: "Trap Disp. Downsample" -> [w1370]
      tunnel: w993 -> [w1368]
      tunnel: w991 -> [w1367]
      tunnel: w990 -> [w1365]
      tunnel: w986 -> [w1364] mode=indexing
      tunnel: [w1363] -> w944 mode=indexing
      tunnel: w946 -> [w1361] mode=indexing
      tunnel: w945 -> [w1359]
      n462 = call "downsample 1D array - double.vi"("Ave N"=w1370, "Array In"=w1371) -> ("Array Out"=w1369:dbl[])  [unwired: 1 out]
      n463 = Subtract(x=w1369, y=w1361) -> (x-y=w1362:dbl[])
      n464 = Multiply(x=w1359, y=w1362) -> (x*y=w1360:dbl[])
      n465 = Bundle By Name("Y"=w1360, "dt"=w1368, "t0"=w1367) -> (w1366:waveform(dbl))  [unwired: 1 out]
      n466 = Set Waveform Attribute(5:w1364, 6:w1365, 7:w1366) -> (3:w1363:waveform(dbl))  [unwired: 1 in, 2 out]
    }
    "Trap Positions" <- w944
    n467 = Bundle("APD 1", "APD 2") -> (w1181:cluster{string, string})  [unwired: 1 out]
    n468 = Cluster To Array(cluster=w1181) -> (array=w1178:string[])
    n469 = for "APD" {
      tunnel: w1149 -> [w2445] mode=indexing
      tunnel: w1018 -> [w2453]
      tunnel: [w2449] -> w1025 mode=indexing
      tunnel: "APD Disp. Scale" -> [w2450]
      tunnel: w990 -> [w2448]
      tunnel: w1178 -> [w2447] mode=indexing
      tunnel: "APD Disp. Downsample" -> [w2443]
      tunnel: [w2446] -> w1177
      workers-P: _ -> [_]
      tunnel: w991 -> [w2442]
      n470 = call "integrate 1D array interval - double.vi"("Ave N"=w2443, "Array In"=w2445) -> ("Array Out"=w2444:dbl[])  [unwired: 1 out]
      n471 = Multiply(x=w2453, y=w2443) -> (x*y=w2446:dbl)
      n472 = Divide(x=w2444, y=w2450) -> (x/y=w2451:dbl[])
      n473 = Bundle By Name("t0"=w2442, "Y"=w2451, "dt"=w2446) -> (w2452:waveform(dbl))  [unwired: 1 out]
      n474 = Set Waveform Attribute(5:w2447, 6:w2448, 7:w2452) -> (3:w2449:waveform(dbl))  [unwired: 1 in, 2 out]
    }
    "APD Display Period (s)" <- w1177
    n475 = Reciprocal(x=w1177) -> (1/x=→"APD Display Freq. (Hz)":dbl)
    n476 = local read "Display Period (s)"() -> (w1053:dbl)
    n477 = Increment(x=w1160) -> (x+1=w1161:dbl)
    n478 = Index Array(array=w944, index=0) -> (element=w942:waveform(dbl))
    n479 = To Double Precision Float(number=w1069) -> (double precision float=w1068:dbl[])
    n480 = feedback #2(w1161) -> (w1164:dbl)
    n481 = Select(t=0, s=w1151, f=w1164) -> (s? t:f=w1157:dbl)
    n482 = Array Size(array=w1068) -> (size(s)=w1163:i32)
    n483 = Add(x=w1163, y=w1157) -> (x+y=w1158:dbl)
    n484 = Unbundle By Name(w942) -> ("Y"=w940:dbl[])
    n485 = feedback #3(w1069) -> (w1147:u32[])
    n486 = Build Array (concatenate)(w1147, w1069) -> (w1144:u32[])
    n487 = feedback #4(w1005) -> (w1024:u32[])
    n488 = Divide(x="Bead Sep. Int. Time (s)", y=w1053) -> (x/y=w938:dbl)
    n489 = Build Array (concatenate)(w1024, w1005) -> (w1023:u32[])
    n490 = Greater?(x=w1158, y=w1160) -> (0:w1159:bool)
    n491 = feedback #5(w940) -> (w941:dbl[])
    n492 = Build Array (concatenate)(w940, w941) -> (w939:dbl[])
    n493 = Select(t=w1157, s=w1159, f=w1158) -> (s? t:f=w1156:dbl)
    n494 = feedback-in #2(w1156) -> ()
    n495 = Array Size(array=w1144) -> (size(s)=w1141:i32)
    n496 = Array Size(array=w1069) -> (size(s)=w1143:i32)
    n497 = local read "MCL Scanning"() -> (w1154:bool)
    n498 = local read "APD Integration Time (s)"() -> (w1032:dbl)
    n499 = Build Array (concatenate)(w1025, w1182) -> (w1027:waveform(dbl)[])
    "All Signals" <- w1027
    n500 = Split 1D Array(array=w939, index=w938) -> (first subarray=w932:dbl[])  [unwired: 1 out]
    n501 = feedback-in #5(w932) -> ()
    n502 = Multiply(x=w1143, y="APD Ave N") -> (x*y=w1142:dbl)
    n503 = Greater?(x=w1141, y=w1142) -> (0:w1145:bool)
    n504 = Not(x=w1159) -> (.not. x?=w1153:bool)
    n505 = To Double Precision Float(number=w1005) -> (double precision float=w1004:dbl[])
    n506 = call <vilib>:"Mean.vi"("X"=w932) -> ("mean"=w931:dbl)  [unwired: 1 out]
    "Mean T1 Position (nm)" <- w931
    n507 = Subtract(x=w932, y=w931) -> (x-y=w937:dbl[])
    n508 = Square(x=w937) -> (x^2=w936:dbl[])
    n509 = And(x=w1153, y=w1154) -> (x .and. y?=w1155:bool)
    n510 = call <vilib>:"Mean.vi"("X"=w936) -> ("mean"=w935:dbl)  [unwired: 1 out]
    n511 = case shown="True" w1145 {
      tunnel: w1144 -> [w2026 w2033]
      tunnel: [w2026 w2031] -> w1085
      tunnel: w1142 -> [_ w2028]
      tunnel: w1141 -> [_ w2032]
      tunnel: w1023 -> [w2025 w2030]
      tunnel: [w2025 w2027] -> w1020
      frame False {
      }
      frame True {
        n512 = Subtract(x=w2032, y=w2028) -> (x-y=w2029:dbl)
        n513 = Array Subset(array=w2033, index=w2029, length=w2028) -> (w2031:u32[])
        n514 = Array Subset(array=w2030, index=w2029, length=w2028) -> (w2027:u32[])
      }
    }
    n515 = feedback-in #3(w1085) -> ()
    n516 = feedback-in #4(w1020) -> ()
    n517 = Or(x=w1155, y=w1151) -> (x .or. y?=w1152:bool)
    n518 = Square Root(x=w935) -> (sqrt(x)=w934:dbl)
    n519 = Equal?(x="Tab Control 6", y=T30."High Res Display") -> (x = y?=w1075:bool)
    n520 = Multiply(x="APD Disp. Scale", y=w1025) -> (x*y=w1034:waveform(dbl)[])
    n521 = Multiply(x="APD Disp. Downsample", y=w1032) -> (x*y=w1030:dbl)
    n522 = Multiply(x=10.0, y=w934) -> (x*y=→"Trap 1 Position RMS (A)":dbl)
    n523 = Divide(x=w1034, y=w1030) -> (x/y=w1002:waveform(dbl)[])
    n524 = Index Array(array=w1002, index=0) -> (element=w1012:waveform(dbl))
    n525 = case "For computing FFTs for display" shown="True" "Compute FFT" {
      tunnel: w1029 -> [_ w3289]
      frame False {
      }
      frame True {
        n526 = Build Array("FFT 1 Choice 1", "FFT 1 Choice 2", "FFT 2 Choice 1", "FFT 2 Choice 2") -> (w3282:u16[])
        n527 = Array Size(array=w3289) -> (size(s)=w3288:i32)
        n528 = feedback-in #6(w3282) -> ()
        n529 = feedback #6(u16[] [100, 100, 100, 100]) -> (w3283:u16[])
        n530 = feedback-in #7("# Spectra to Ave.") -> ()
        n531 = feedback #7("# Spectra to Ave.") -> (w3280:dbl)
        n532 = Not Equal?(x="# Spectra to Ave.", y=w3280) -> (x != y?=w3279:bool)
        n533 = Not Equal?(x=w3282, y=w3283) -> (x != y?=w3281:bool)
        n534 = feedback #8(1.0) -> (w3266:dbl)
        n535 = Compound Arithmetic op=OR("Reset FFT", w3281, w3279) -> (w3264:bool)
        n536 = Select(t=1.0, s=w3264, f=w3266) -> (s? t:f=w3268:dbl)
        n537 = Greater?(x=w3268, y="# Spectra to Ave.") -> (0:w3287:bool)
        n538 = Increment(x=w3268) -> (x+1=w3267:dbl)
        n539 = feedback-in #8(w3267) -> ()
        n540 = local read "DMA Update Period (s)"() -> (w3262:dbl)
        n541 = Multiply(x="# Spectra to Ave.", y=w3262) -> (x*y=→"Ave. Time (s)":dbl)
        n542 = Build Array(cluster{"f0":dbl, "df":dbl, "magnitude":dbl[]} {"f0"=0.0, "df"=0.0, "magnitude"=[]} ("PSD")) -> (w3271:cluster{"f0":dbl, "df":dbl, "magnitude":dbl[]}[])
        n543 = Build Array(w3271, w3271, w3271, w3271) -> (w3273:T44)
        n544 = feedback #9(w3273) -> (w3278:T44)
        n545 = for {
          N: 4 -> [_]
          tunnel: w3282 -> [w3311] mode=indexing
          tunnel: w3289 -> [w3312]
          tunnel: w3288 -> [w3314]
          tunnel: w3264 -> [w3307]
          tunnel: w3287 -> [w3306]
          tunnel: "# Spectra to Ave." -> [w3305]
          tunnel: [w3304] -> w3277 mode=indexing
          tunnel: w3278 -> [w3309] mode=indexing
          tunnel: [w3308] -> w3265 mode=indexing
          tunnel: w3268 -> [w3303]
          n546 = Less?(x=w3311, y=w3314) -> (x < y?=w3313:bool)
          n547 = Index Array(array=w3312, index=w3311) -> (element=w3310:waveform(dbl))
          n548 = case shown="True" w3313 {
            tunnel: w3310 -> [_ w3331]
            tunnel: w3309 -> [w3316 w3329]
            tunnel: [w3316 w3317] -> w3308
            tunnel: w3307 -> [_ w3328]
            tunnel: w3306 -> [_ w3321]
            tunnel: w3305 -> [_ w3320]
            tunnel: [cluster{"f0":dbl, "df":dbl, "magnitude":dbl[]} {"f0"=0.0, "df"=0.0, "magnitude"=[]} ("PSD") w3322] -> w3304
            tunnel: w3303 -> [_ w3319]
            frame False {
            }
            frame True {
              n549 = call <vilib>:"Std Deviation and Variance.vi"("X"=w3331) -> ("mean"=w3332:dbl)  [unwired: 1 in, 2 out]
              n550 = Subtract(x=w3331, y=w3332) -> (x-y=w3330:waveform(dbl))
              n551 = xnode "Spectral Measurements"("Signals"=w3330) -> ("PSD"=w3324:cluster{"f0":dbl, "df":dbl, "magnitude":dbl[]})  [unwired: 1 in, 1 out]
              n552 = case shown="False" w3328 {
                tunnel: w3329 -> [w3341 _]
                tunnel: [w3337 w3346] -> w3317
                tunnel: w3324 -> [w3340 w3347]
                tunnel: w3321 -> [w3339 _]
                frame False {
                  n553 = Build Array (concatenate)(w3341, w3340) -> (w3338:cluster{"f0":dbl, "df":dbl, "magnitude":dbl[]}[])
                  n554 = case shown="True" w3339 {
                    tunnel: w3338 -> [w3342 w3345]
                    tunnel: [w3342 w3343] -> w3337
                    frame False {
                    }
                    frame True {
                      n555 = Delete From Array(array=w3345, index=0) -> (array with subset deleted=w3343:cluster{"f0":dbl, "df":dbl, "magnitude":dbl[]}[])  [unwired: 1 in, 1 out]
                    }
                  }
                }
                frame True {
                  n556 = Build Array(w3347) -> (w3346:cluster{"f0":dbl, "df":dbl, "magnitude":dbl[]}[])
                }
              }
              n557 = for {
                tunnel: w3317 -> [w3336] mode=indexing
                tunnel: [w3335] -> w3327 mode=indexing
                workers-P: _ -> [_]
                n558 = Unbundle By Name(w3336) -> ("magnitude"=w3335:dbl[])
              }
              n559 = Transpose 2D Array(2D array=w3327) -> (transposed array=w3326:dbl[][])
              n560 = for {
                tunnel: w3326 -> [w3334] mode=indexing
                tunnel: [w3333] -> w3325 mode=indexing
                workers-P: _ -> [_]
                n561 = Add Array Elements(numeric array=w3334) -> (sum=w3333:dbl)
              }
              n562 = Select(t=w3320, s=w3321, f=w3319) -> (s? t:f=w3318:dbl)
              n563 = Divide(x=w3325, y=w3318) -> (x/y=w3323:dbl[])
              n564 = Bundle By Name(cluster=w3324, "magnitude"=w3323) -> (w3322:cluster{"f0":dbl, "df":dbl, "magnitude":dbl[]})
            }
          }
        }
        n565 = case shown="True" w3264 {
          tunnel: w3265 -> [w3296 w3302]